vi "1_ScanCameraFocus.vi"() -> ()   [LabVIEW 2016]
uses:
  <vilib>/vision/driver/NI_Vision_Acquisition_Software.lvlib
  <vilib>/vision/NI_Vision_Development_Module.lvlib
panel:
  out "Z step":dbl=12.0
  out "Image":T1(plugin-control)
  in  "End Z [mm]":dbl=10.0
  in  "Stepsize [mm]":dbl=0.1
  in  "Match parameters":T2={"Number of Matches Requested"=10, "Minimum Match Score"=500.0, "Angle Ranges"=[]}
  in  "Template File Path":path=path "E:/XYZstage+Camera_CollectedImages/12-14-2016/test_sub_highVoltageContact_-23,-32,3.png"
  in  "Axes Speeds [mm/s]":T3={"X Speed"=25.0, "Y Speed"=3.0, "Z Speed"=1.0}
  in  "Initial Location [mm]":T4={"Go to X"=-23.0, "Go to Y"=-32.0, "Go to Z"=-2.0}
  out "Moving":bool
  out "XYZ Stage Current Position":T5={"X [-750, 750 mm]"=-23.00047348022461, "Y [-150, 30 mm]"=-32.00033050537109, "Z [-50, 50 mm]"=10.000400000000003}
  out "Error report":errorcluster
  in  "Camera Name":refnum<k21>="cam0" caption="IMAQdx Session"
  # "ANALYSIS"
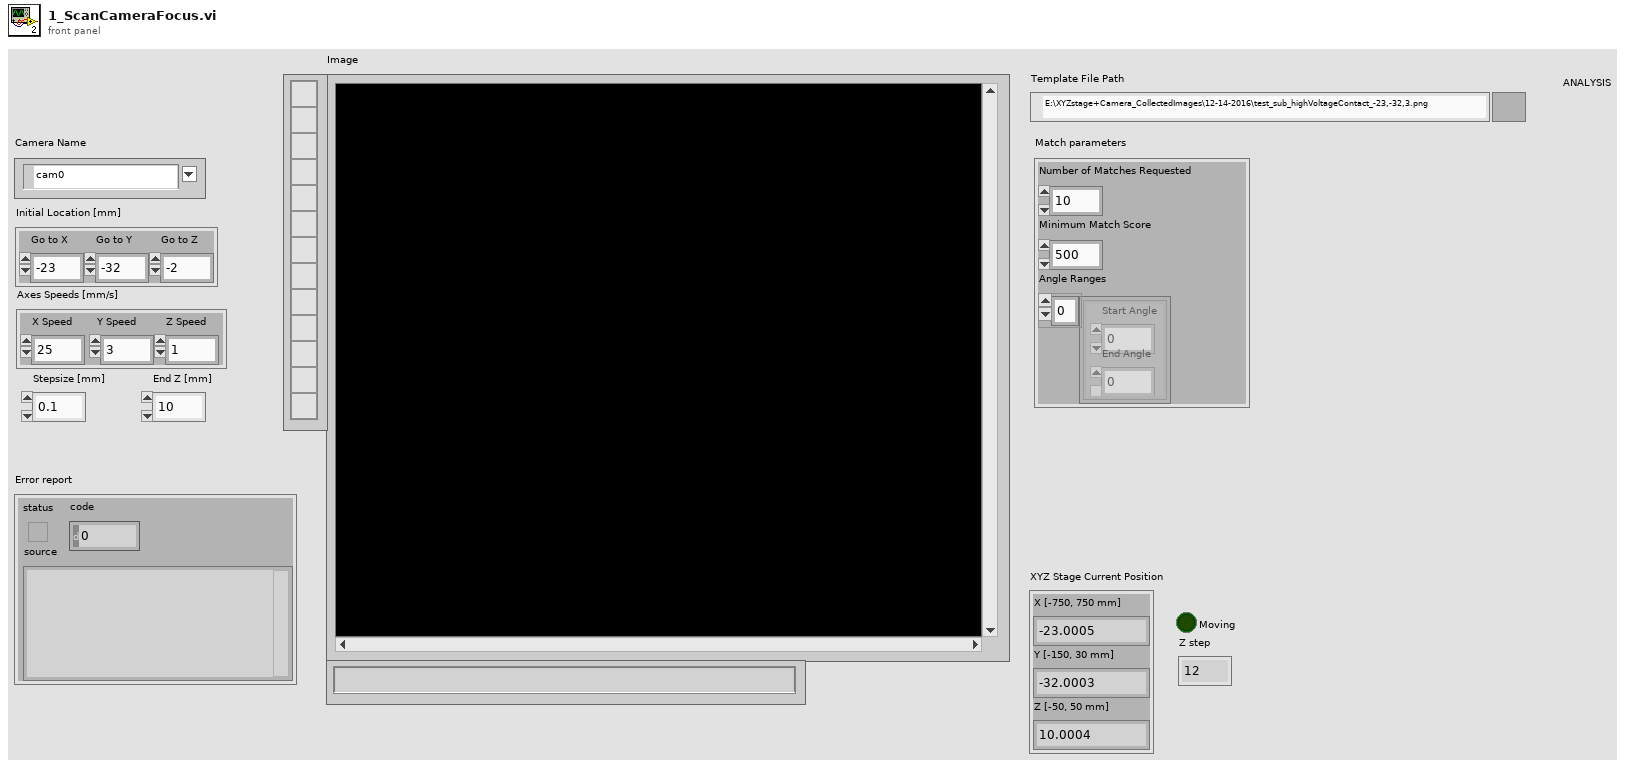
[diagram p1: front panel]
types:
  T1 = typedef "IMAQ Image.ctl" = refnum<image>
  T2 = cluster{"Number of Matches Requested":i32, "Minimum Match Score":sgl, "Angle Ranges":cluster{"Start Angle":sgl, "End Angle":sgl}[]}
  T3 = cluster{"X Speed":dbl, "Y Speed":dbl, "Z Speed":dbl}
  T4 = cluster{"Go to X":dbl, "Go to Y":dbl, "Go to Z":dbl}
  T5 = cluster{"X [-750, 750 mm]":dbl, "Y [-150, 30 mm]":dbl, "Z [-50, 50 mm]":dbl}
  T6 = typedef "Image Type" = u32
  T7 = typedef "IMAQdx.ctl" = refnum<k21>
  T8 = cluster{"Final X":dbl, "Final Y":dbl, "Final Z":dbl}
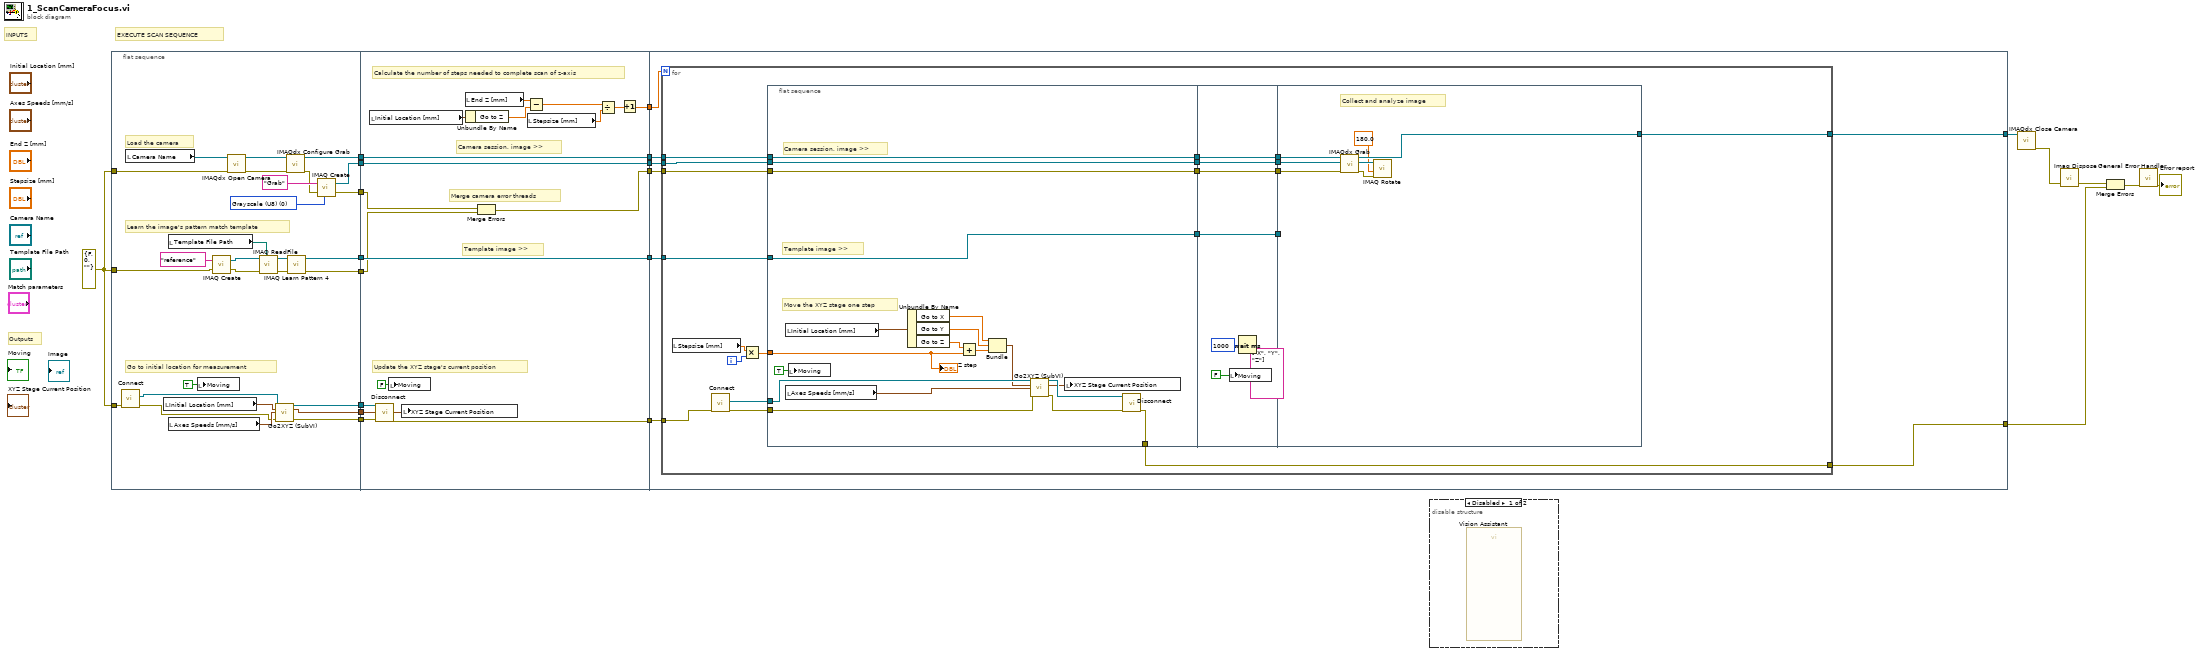
[diagram p0: block diagram]
diagram:
  w1 = errorcluster {"status"=FALSE, "code"=0, "source"=""} ("error in (no error)")
  # "EXECUTE SCAN SEQUENCE"
  # "Outputs"
  # "INPUTS"
  n1 = flat-sequence {
    tunnel: [w49] -> w17
    tunnel: [w48] -> w16
    tunnel: [w43] -> w15
    tunnel: [w32] -> w11
    tunnel: [w28] -> w10
    tunnel: [w27] -> w8
    tunnel: [w26] -> w5
    tunnel: [w25] -> w4
    tunnel: w1 -> [w24]
    tunnel: w1 -> [w23]
    tunnel: w1 -> [w22]
    tunnel: w17 -> [w62]
    tunnel: w16 -> [w61]
    tunnel: w15 -> [w66]
    tunnel: [w50] -> w14
    tunnel: [w60] -> w13
    tunnel: [w58] -> w12
    tunnel: w11 -> [w58]
    tunnel: w10 -> [w57]
    tunnel: [w57] -> w9
    tunnel: w8 -> [w55]
    tunnel: [w53] -> w7
    tunnel: [w56] -> w6
    tunnel: w5 -> [w56]
    tunnel: w4 -> [w54]
    tunnel: w14 -> [w68]
    tunnel: w13 -> [w75]
    tunnel: w12 -> [w74]
    tunnel: w9 -> [w73]
    tunnel: w7 -> [w72]
    tunnel: w6 -> [w71]
    tunnel: [w70] -> w3
    tunnel: [w69] -> w2
    frame #0 {
      w30 = T6 0 items=["Grayscale (U8)", "Grayscale (I16)", "Grayscale (SGL)", "Complex (CSG)", "RGB (U32)", "HSL (U32)", "RGB (U64)", "Grayscale (U16)"] ("Image Type")
      # "Learn the image's pattern match template"
      # "Load the camera"
      # "Go to initial location for measurement"
      n2 = call "Connect.vi"("error in (no error)"=w22) -> ("error out"=w42:errorcluster, "controller"=w44:refnum<k24>)  [unwired: 9 in]
      n3 = local read "Camera Name"() -> (w41:refnum<k21>)
      n4 = local read "Initial Location [mm]"() -> (w45:T4)
      n5 = local read "Template File Path"() -> (w38:path)
      n6 = local read "Axes Speeds [mm/s]"() -> (w46:T3)
      n7 = local write "Moving"(TRUE ("Moving")) -> ()
      n8 = call "IMAQ Create"("Image Name"="reference", "error in (no error)"=w24) -> ("New Image"=w37:T1, "error out"=w36:errorcluster)  [unwired: 3 in]
      n9 = call <vilib>:"IMAQdx Open Camera.vi"("error in"=w23, "Session In"=w41) -> ("error out"=w39:errorcluster, "Session Out"=w40:T7)  [unwired: 1 in, 7 out]
      n10 = call "IMAQ ReadFile"("File Path"=w38, "error in (no error)"=w36, "Image"=w37) -> ("error out"=w33:errorcluster, "Image Out"=w34:T1)  [unwired: 4 in, 3 out]
      n11 = call "Go2XYZ (SubVI).vi"(".NET Refnum in"=w44, "Go to Coordinates"=w45, "Axis Speeds"=w46, "error in (no error)"=w42) -> (".NET Refnum out"=w49:refnum<k24>, "Final Position"=w43:T8, "error out"=w48:errorcluster)  [unwired: 8 in, 1 out]
      n12 = call <vilib>:"IMAQdx Configure Grab.vi"("error in"=w39, "Session In"=w40) -> ("error out"=w29:errorcluster, "Session Out"=w32:T7)  [unwired: 8 out]
      n13 = call "IMAQ Learn Pattern 4"("error in (no error)"=w33, "Image"=w34) -> ("error out"=w25:errorcluster, "Template Image Out"=w26:T1)  [unwired: 7 in, 1 out]
      n14 = call "IMAQ Create"("Image Name"="Grab", "Image Type"=w30, "error in (no error)"=w29) -> ("New Image"=w28:T1, "error out"=w27:errorcluster)  [unwired: 1 in, 1 out]
    }
    frame #1 {
      # "Merge camera error threads"
      # "Camera session, image >>"
      # "Template image >>"
      # "Calculate the number of steps needed to complete scan of z-axis"
      # "Update the XYZ stage's current position"
      n15 = local read "Initial Location [mm]"() -> (w65:T4)
      n16 = call "Disconnect.vi"("error in (no error)"=w61, "controller"=w62) -> ("error out"=w60:errorcluster)  [unwired: 9 in]
      n17 = local write "Moving"(FALSE ("Moving")) -> ()
      n18 = local write "XYZ Stage Current Position"(w66) -> ()
      n19 = local read "End Z [mm]"() -> (w52:dbl)
      n20 = Unbundle By Name(w65) -> ("Go to Z"=w64:dbl)
      n21 = Merge Errors(w55, w54) -> (w53:errorcluster)
      n22 = Subtract(x=w52, y=w64) -> (x-y=w63:dbl)
      n23 = local read "Stepsize [mm]"() -> (w59:dbl)
      n24 = Divide(x=w63, y=w59) -> (x/y=w51:dbl)
      n25 = Increment(x=w51) -> (x+1=w50:dbl)
    }
    frame #2 {
      n26 = for {
        N: w68 -> [_]
        tunnel: w75 -> [w92]
        tunnel: w74 -> [w89]
        tunnel: w73 -> [w88]
        tunnel: w72 -> [w87]
        tunnel: w71 -> [w86]
        tunnel: [w85] -> w70
        tunnel: [w84] -> w69
        i -> [w94]
        (unwired) string[] ["X", "Y", "Z"] ("Axes Names")
        n27 = local read "Stepsize [mm]"() -> (w91:dbl)
        n28 = call "Connect.vi"("error in (no error)"=w92) -> ("error out"=w90:errorcluster, "controller"=w95:refnum<k24>)  [unwired: 9 in]
        n29 = Multiply(x=w91, y=w94) -> (x*y=w93:dbl)
        n30 = flat-sequence {
          tunnel: w95 -> [w114]
          tunnel: w90 -> [w113]
          tunnel: w93 -> [w108]
          tunnel: [w100] -> w83
          tunnel: w89 -> [w100]
          tunnel: w88 -> [w99]
          tunnel: [w99] -> w81
          tunnel: w87 -> [w98]
          tunnel: [w98] -> w79
          tunnel: [w97] -> w77
          tunnel: w86 -> [w97]
          tunnel: [w96] -> w85
          tunnel: w83 -> [w120]
          tunnel: [w120] -> w82
          tunnel: w81 -> [w119]
          tunnel: [w119] -> w80
          tunnel: w79 -> [w118]
          tunnel: [w118] -> w78
          tunnel: w77 -> [w117]
          tunnel: [w117] -> w76
          tunnel: w82 -> [w127]
          tunnel: w80 -> [w126]
          tunnel: w78 -> [w125]
          tunnel: w76 -> [_]
          tunnel: [w124] -> w84
          frame #0 {
            # "Camera session, image >>"
            # "Template image >>"
            # "Move the XYZ stage one step"
            n31 = local read "Initial Location [mm]"() -> (w110:T4)
            n32 = local read "Axes Speeds [mm/s]"() -> (w111:T3)
            n33 = local write "Moving"(TRUE ("Moving")) -> ()
            n34 = Unbundle By Name(w110) -> ("Go to X"=w105:dbl, "Go to Y"=w106:dbl, "Go to Z"=w109:dbl)
            n35 = Add(x=w109, y=w108) -> (x+y=w107:dbl)
            n36 = Bundle("Go to X"=w105, "Go to Y"=w106, w107) -> (w104:cluster{"Go to X":dbl, "Go to Y":dbl, dbl})  [unwired: 1 in]
            n37 = call "Go2XYZ (SubVI).vi"(".NET Refnum in"=w114, "Go to Coordinates"=w104, "Axis Speeds"=w111, "error in (no error)"=w113) -> (".NET Refnum out"=w103:refnum<k24>, "Final Position"=w101:T8, "error out"=w102:errorcluster)  [unwired: 8 in, 1 out]
            n38 = local write "XYZ Stage Current Position"(w101) -> ()
            n39 = call "Disconnect.vi"("error in (no error)"=w102, "controller"=w103) -> ("error out"=w96:errorcluster)  [unwired: 9 in]
            "Z step" <- w108
          }
          frame #1 {
            n40 = local write "Moving"(FALSE ("Moving")) -> ()
            n41 = Wait (ms)(milliseconds to wait=u32 1000) -> ()  [unwired: 1 out]
          }
          frame #2 {
            # "Collect and analyze image"
            n42 = call <vilib>:"IMAQdx Grab.vi"("error in"=w125, "Image In"=w126, "Session In"=w127) -> ("error out"=w122:errorcluster, "Image Out"=w123:T1, "Session Out"=w124:T7)  [unwired: 1 in, 5 out]
            n43 = call "IMAQ Rotate"("error in (no error)"=w122, "Angle (degrees)"=sgl 180.0, "Image Src"=w123) -> ()  [unwired: 7 in, 2 out]
          }
        }
      }
    }
  }
  n44 = disable-structure shown="Disabled" {
    frame Disabled {
      n45 = call "Vision Assistant"() -> ()  [unwired: 25 in, 3 out]
    }
    frame Enabled {
    }
  }
  n46 = call <vilib>:"IMAQdx Close Camera.vi"("Session In"=w2) -> ("error out"=w20:errorcluster)  [unwired: 1 in, 9 out]
  n47 = call "Imaq Dispose"("error in (no error)"=w20) -> ("error out"=w19:errorcluster)  [unwired: 5 in]
  n48 = Merge Errors(w19, w3) -> (w18:errorcluster)
  n49 = call <vilib>:"General Error Handler.vi"("error in (no error)"=w18) -> ("error out"=→"Error report":errorcluster)  [unwired: 2 in, 12 out]
